vi "Dresden R2R Sputter 03.02.2018 IY24.vi"() -> ()   [LabVIEW 2009] (continued)
                                stop <- w22715 stop-if-true
                                n21716 = Greater?(x=w22721, y=50) -> (0:w22719:bool)
                                n21717 = case shown="True" w22719 {
                                frame #0 {
                                }
                                frame #1 {
                                n21718 = local write "Semi"(TRUE ("Semi")) -> ()
                                n21719 = local write "Error Message"("Start up process  cancelled\nbecause MP not stopped.\nPlease check MP4 connections." ("Error Message")) -> ()
                                }
                                }
                                n21720 = local read "Ch4_Mp_di"() -> (w22718:bool)
                                n21721 = case shown="True" w22718 {
                                tunnel: [TRUE FALSE] -> w22717
                                frame #0 {
                                }
                                frame #1 {
                                n21722 = Wait Until Next ms Multiple(millisecond multiple=u32 200) -> ()  [unwired: 1 out]
                                n21723 = local write "Ch4_Mp_do"(FALSE ("Ch1_Tp_bv_do")) -> ()
                                }
                                }
                                n21724 = local read "Semi"() -> (w22716:bool)
                                n21725 = Or(x=w22717, y=w22716) -> (x .or. y?=w22715:bool)
                                }
                                }
                                frame #1 {
                                }
                                }
                                }
                                frame #1 {
                                n21726 = local read "Semi"() -> (w22728:bool)
                                n21727 = case shown="False" w22728 {
                                frame #0 {
                                n21728 = local write "Ch4_PA10"(TRUE ("PA3")) -> ()
                                n21729 = Wait Until Next ms Multiple(millisecond multiple=u32 1000) -> ()  [unwired: 1 out]
                                }
                                frame #1 {
                                }
                                }
                                }
                                }
                              }
                              frame #1 {
                              }
                            }
                          }
                          frame #6 {
                            # "OPEN PL-VBV1"
                            n21730 = local read "Semi"() -> (w22731:bool)
                            n21731 = case shown="False" w22731 {
                              frame #0 {
                                n21732 = stacked-sequence {
                                frame #0 {
                                n21733 = local read "Semi"() -> (w22732:bool)
                                n21734 = case shown="False" w22732 {
                                frame #0 {
                                n21735 = while {
                                i -> [w22739]
                                stop <- w22734 stop-if-true
                                n21736 = Greater?(x=w22739, y=50) -> (0:w22737:bool)
                                n21737 = case shown="True" w22737 {
                                frame #0 {
                                }
                                frame #1 {
                                n21738 = local write "Semi"(TRUE ("Semi")) -> ()
                                n21739 = local write "Error Message"("Start up process  cancelled\nbecause  PL-VBV not opened.\nPlease check PL-VBV4 connections." ("Error Message")) -> ()
                                }
                                }
                                n21740 = local read "Ch4_Pl_atm_di"() -> (w22733:bool)
                                n21741 = case shown="False" w22733 {
                                tunnel: [w22741 TRUE] -> w22736
                                frame #0 {
                                n21742 = local read "Ch4_Pl_vbv_di"() -> (w22740:bool)
                                n21743 = case shown="False" w22740 {
                                tunnel: [FALSE TRUE] -> w22741
                                frame #0 {
                                n21744 = local write "Ch4_Pl_vbv_do"(TRUE ("Ch1_Tp_bv_do")) -> ()
                                n21745 = Wait Until Next ms Multiple(millisecond multiple=u32 200) -> ()  [unwired: 1 out]
                                }
                                frame #1 {
                                }
                                }
                                }
                                frame #1 {
                                }
                                }
                                n21746 = local read "Semi"() -> (w22735:bool)
                                n21747 = Or(x=w22736, y=w22735) -> (x .or. y?=w22734:bool)
                                }
                                }
                                frame #1 {
                                }
                                }
                                }
                                frame #1 {
                                n21748 = local read "Semi"() -> (w22749:bool)
                                n21749 = case shown="False" w22749 {
                                frame #0 {
                                n21750 = local write "Ch4_PA11"(TRUE ("PA3")) -> ()
                                n21751 = Wait Until Next ms Multiple(millisecond multiple=u32 1000) -> ()  [unwired: 1 out]
                                }
                                frame #1 {
                                }
                                }
                                }
                                }
                              }
                              frame #1 {
                              }
                            }
                          }
                          frame #7 {
                            # "CHECK PL-PRESSURE"
                            n21752 = local read "Semi"() -> (w22752:bool)
                            n21753 = case shown="False" w22752 {
                              frame #0 {
                                n21754 = stacked-sequence {
                                frame #0 {
                                n21755 = local read "Semi"() -> (w22753:bool)
                                n21756 = case shown="False" w22753 {
                                frame #0 {
                                n21757 = while {
                                i -> [w22760]
                                stop <- w22755 stop-if-true
                                n21758 = Greater?(x=w22760, y=50) -> (0:w22758:bool)
                                n21759 = case shown="True" w22758 {
                                frame #0 {
                                }
                                frame #1 {
                                n21760 = local write "Semi"(TRUE ("Semi")) -> ()
                                n21761 = local write "Error Message"("Start up process  cancelled\nbecause  PL-ATM not opened.\nPlease check PL-ATM connections." ("Error Message")) -> ()
                                }
                                }
                                n21762 = local read "Ch4_Pl_atm_di"() -> (w22754:bool)
                                n21763 = case shown="True" w22754 {
                                tunnel: [FALSE TRUE] -> w22757
                                frame #0 {
                                }
                                frame #1 {
                                n21764 = Wait Until Next ms Multiple(millisecond multiple=u32 500) -> ()  [unwired: 1 out]
                                }
                                }
                                n21765 = local read "Semi"() -> (w22756:bool)
                                n21766 = Or(x=w22757, y=w22756) -> (x .or. y?=w22755:bool)
                                }
                                }
                                frame #1 {
                                }
                                }
                                }
                                frame #1 {
                                n21767 = local read "Semi"() -> (w22766:bool)
                                n21768 = case shown="False" w22766 {
                                frame #0 {
                                n21769 = local write "Ch4_PA12"(TRUE ("PA3")) -> ()
                                n21770 = Wait Until Next ms Multiple(millisecond multiple=u32 1000) -> ()  [unwired: 1 out]
                                }
                                frame #1 {
                                }
                                }
                                }
                                }
                              }
                              frame #1 {
                              }
                            }
                          }
                          frame #8 {
                            # "False CH-ATM"
                            n21771 = local read "Semi"() -> (w22769:bool)
                            n21772 = case shown="False" w22769 {
                              frame #0 {
                                n21773 = stacked-sequence {
                                frame #0 {
                                n21774 = local read "Semi"() -> (w22770:bool)
                                n21775 = case shown="False" w22770 {
                                frame #0 {
                                n21776 = local write "Ch4_Ch_atm_do"(FALSE ("Ch1_Pl_atm_do")) -> ()
                                }
                                frame #1 {
                                }
                                }
                                }
                                frame #1 {
                                n21777 = local read "Semi"() -> (w22772:bool)
                                n21778 = case shown="False" w22772 {
                                frame #0 {
                                n21779 = local write "Ch4_PA13"(TRUE ("PA3")) -> ()
                                n21780 = Wait Until Next ms Multiple(millisecond multiple=u32 1000) -> ()  [unwired: 1 out]
                                }
                                frame #1 {
                                }
                                }
                                }
                                }
                              }
                              frame #1 {
                              }
                            }
                          }
                          frame #9 {
                            # "OPEN PC-BV"
                            n21781 = local read "Semi"() -> (w22775:bool)
                            n21782 = case shown="False" w22775 {
                              frame #0 {
                                n21783 = stacked-sequence {
                                frame #0 {
                                n21784 = local read "Semi"() -> (w22776:bool)
                                n21785 = case shown="False" w22776 {
                                frame #0 {
                                n21786 = stacked-sequence {
                                frame #0 {
                                n21787 = local read "Semi"() -> (w22777:bool)
                                n21788 = case shown="False" w22777 {
                                frame #0 {
                                n21789 = local write "Pc_bv4_auto_open"(TRUE ("Tp1_auto_start")) -> ()
                                }
                                frame #1 {
                                }
                                }
                                }
                                frame #1 {
                                n21790 = local read "Semi"() -> (w22779:bool)
                                n21791 = case shown="False" w22779 {
                                frame #0 {
                                n21792 = Wait (ms)(milliseconds to wait=u32 1000) -> ()  [unwired: 1 out]
                                }
                                frame #1 {
                                }
                                }
                                }
                                frame #2 {
                                n21793 = local read "Semi"() -> (w22781:bool)
                                n21794 = case shown="False" w22781 {
                                frame #0 {
                                n21795 = while {
                                i -> [w22787]
                                stop <- w22783 stop-if-true
                                n21796 = local read "Pc_bv_opened_ch4"() -> (w22785:bool)
                                n21797 = Greater?(x=w22787, y=120) -> (0:w22786:bool)
                                n21798 = local read "Semi"() -> (w22784:bool)
                                n21799 = Compound Arithmetic op=OR(w22784, w22785, w22786) -> (w22783:bool)
                                n21800 = Wait (ms)(milliseconds to wait=u32 500) -> ()  [unwired: 1 out]
                                }
                                }
                                frame #1 {
                                }
                                }
                                }
                                frame #3 {
                                n21801 = local read "Semi"() -> (w22789:bool)
                                n21802 = case shown="False" w22789 {
                                frame #0 {
                                n21803 = local read "Pc_bv_opened_ch4"() -> (w22790:bool)
                                n21804 = case shown="False" w22790 {
                                frame #0 {
                                n21805 = local write "Pc_bv4_auto_open"(TRUE ("Pc_bv1_auto_open")) -> ()
                                }
                                frame #1 {
                                }
                                }
                                }
                                frame #1 {
                                }
                                }
                                }
                                frame #4 {
                                n21806 = local read "Semi"() -> (w22792:bool)
                                n21807 = case shown="False" w22792 {
                                frame #0 {
                                n21808 = local read "Pc_bv_opened_ch4"() -> (w22793:bool)
                                n21809 = case shown="False" w22793 {
                                frame #0 {
                                n21810 = Wait (ms)(milliseconds to wait=u32 1000) -> ()  [unwired: 1 out]
                                }
                                frame #1 {
                                }
                                }
                                }
                                frame #1 {
                                }
                                }
                                }
                                frame #5 {
                                n21811 = local read "Semi"() -> (w22795:bool)
                                n21812 = case shown="False" w22795 {
                                frame #0 {
                                n21813 = while {
                                i -> [w22801]
                                stop <- w22797 stop-if-true
                                n21814 = local read "Pc_bv_opened_ch4"() -> (w22799:bool)
                                n21815 = Greater?(x=w22801, y=120) -> (0:w22800:bool)
                                n21816 = local read "Semi"() -> (w22798:bool)
                                n21817 = Compound Arithmetic op=OR(w22798, w22799, w22800) -> (w22797:bool)
                                n21818 = Wait (ms)(milliseconds to wait=u32 500) -> ()  [unwired: 1 out]
                                }
                                }
                                frame #1 {
                                }
                                }
                                }
                                frame #6 {
                                n21819 = local read "Semi"() -> (w22803:bool)
                                n21820 = case shown="False" w22803 {
                                frame #0 {
                                n21821 = local read "Pc_bv_opened_ch4"() -> (w22804:bool)
                                n21822 = case shown="False" w22804 {
                                frame #0 {
                                n21823 = local write "Error Message"("Start up process  cancelled\nbecause  PC-BV not opened.\nPlease check PC-BV4 connections." ("Error Message")) -> ()
                                n21824 = Wait (ms)(milliseconds to wait=u32 1000) -> ()  [unwired: 1 out]
                                }
                                frame #1 {
                                }
                                }
                                }
                                frame #1 {
                                }
                                }
                                }
                                }
                                }
                                frame #1 {
                                }
                                }
                                }
                                frame #1 {
                                n21825 = local read "Semi"() -> (w22807:bool)
                                n21826 = case shown="False" w22807 {
                                frame #0 {
                                n21827 = Wait Until Next ms Multiple(millisecond multiple=u32 1000) -> ()  [unwired: 1 out]
                                n21828 = local write "Ch4_PA14"(TRUE ("PA3")) -> ()
                                }
                                frame #1 {
                                }
                                }
                                }
                                }
                              }
                              frame #1 {
                              }
                            }
                          }
                          frame #10 {
                            # "OPEN CH-VBV"
                            n21829 = local read "Semi"() -> (w22810:bool)
                            n21830 = case shown="False" w22810 {
                              frame #0 {
                                n21831 = stacked-sequence {
                                frame #0 {
                                n21832 = local read "Semi"() -> (w22811:bool)
                                n21833 = case shown="False" w22811 {
                                frame #0 {
                                n21834 = while {
                                i -> [w22818]
                                stop <- w22813 stop-if-true
                                n21835 = Greater?(x=w22818, y=200) -> (0:w22816:bool)
                                n21836 = case shown="True" w22816 {
                                frame #0 {
                                }
                                frame #1 {
                                n21837 = local write "Semi"(TRUE ("Semi")) -> ()
                                n21838 = local write "Error Message"("Start up process  cancelled\nbecause  CH-VBV not opened.\nPlease check  CH-VBV connections." ("Error Message")) -> ()
                                }
                                }
                                n21839 = local read "Ch4_Ch_atm_di"() -> (w22812:bool)
                                n21840 = case shown="False" w22812 {
                                tunnel: [w22819 TRUE] -> w22815
                                frame #0 {
                                n21841 = local read "Ch4_Ch_vbv_di"() -> (w22820:bool)
                                n21842 = case shown="False" w22820 {
                                tunnel: [FALSE TRUE] -> w22819
                                frame #0 {
                                n21843 = local write "Ch4_Ch_vbv_do"(TRUE ("Ch1_Tp_bv_do")) -> ()
                                n21844 = Wait Until Next ms Multiple(millisecond multiple=u32 200) -> ()  [unwired: 1 out]
                                }
                                frame #1 {
                                }
                                }
                                }
                                frame #1 {
                                }
                                }
                                n21845 = local read "Semi"() -> (w22814:bool)
                                n21846 = Or(x=w22815, y=w22814) -> (x .or. y?=w22813:bool)
                                }
                                }
                                frame #1 {
                                }
                                }
                                }
                                frame #1 {
                                n21847 = local read "Semi"() -> (w22828:bool)
                                n21848 = case shown="False" w22828 {
                                frame #0 {
                                n21849 = local write "Ch4_PA15"(TRUE ("PA3")) -> ()
                                n21850 = Wait Until Next ms Multiple(millisecond multiple=u32 1000) -> ()  [unwired: 1 out]
                                }
                                frame #1 {
                                }
                                }
                                }
                                }
                              }
                              frame #1 {
                              }
                            }
                          }
                          frame #11 {
                            # "OPEN/CLOSE TRNS GV-BP"
                            n21851 = local read "Semi"() -> (w22831:bool)
                            n21852 = case shown="False" w22831 {
                              frame #0 {
                                n21853 = stacked-sequence {
                                frame #0 {
                                n21854 = local read "Semi"() -> (w22832:bool)
                                n21855 = case shown="False" w22832 {
                                frame #0 {
                                n21856 = while {
                                i -> [w22841]
                                stop <- w22836 stop-if-true
                                n21857 = Greater?(x=w22841, y=800) -> (0:w22839:bool)
                                n21858 = case shown="True" w22839 {
                                frame #0 {
                                }
                                frame #1 {
                                n21859 = local read "Ch3_pressure"() -> (w22861:dbl)
                                n21860 = Less?(x=w22861, y=1) -> (x < y?=w22860:bool)
                                n21861 = case shown="True" w22860 {
                                frame #0 {
                                n21862 = local write "Error Message"("Start up process  cancelled\nbecause \n Trns GV-BP not closed.\nPlease check \nTrns GV-BP connections." ("Error Message")) -> ()
                                }
                                frame #1 {
                                n21863 = local write "Error Message"("Start up process  cancelled\nbecause \n Trns GV-BP not opened.\nPlease check \nTrns GV-BP connections." ("Error Message")) -> ()
                                }
                                }
                                n21864 = local write "Semi"(TRUE ("Semi")) -> ()
                                }
                                }
                                n21865 = local read "Ch3_pressure"() -> (w22835:dbl)
                                n21866 = Less?(x=w22835, y=1) -> (x < y?=w22833:bool)
                                n21867 = case shown="True" w22833 {
                                tunnel: [w22843 w22851] -> w22838
                                frame #0 {
                                n21868 = local read "Ch4_Trns_gv_bp_di"() -> (w22842:bool)
                                n21869 = case shown="True" w22842 {
                                tunnel: [TRUE FALSE] -> w22843
                                frame #0 {
                                }
                                frame #1 {
                                n21870 = local write "Ch4_Trns_gv_bp_do"(FALSE ("Ch1_Tp_bv_do")) -> ()
                                n21871 = Wait Until Next ms Multiple(millisecond multiple=u32 200) -> ()  [unwired: 1 out]
                                }
                                }
                                }
                                frame #1 {
                                n21872 = local read "Ch4pressure"() -> (w22850:dbl)
                                n21873 = Greater Or Equal?(x=w22850, y=700.0) -> (x >= y?=w22848:bool)
                                n21874 = case shown="True" w22848 {
                                tunnel: [FALSE w22855] -> w22851
                                frame #0 {
                                n21875 = Wait Until Next ms Multiple(millisecond multiple=u32 500) -> ()  [unwired: 1 out]
                                }
                                frame #1 {
                                n21876 = local read "Ch4_Trns_gv_bp_di"() -> (w22854:bool)
                                n21877 = case shown="False" w22854 {
                                tunnel: [FALSE TRUE] -> w22855
                                frame #0 {
                                n21878 = local write "Ch4_Trns_gv_bp_do"(TRUE ("Ch1_Tp_bv_do")) -> ()
                                n21879 = Wait Until Next ms Multiple(millisecond multiple=u32 200) -> ()  [unwired: 1 out]
                                }
                                frame #1 {
                                }
                                }
                                }
                                }
                                }
                                }
                                n21880 = local read "Semi"() -> (w22837:bool)
                                n21881 = Or(x=w22838, y=w22837) -> (x .or. y?=w22836:bool)
                                }
                                }
                                frame #1 {
                                }
                                }
                                }
                                frame #1 {
                                n21882 = local read "Semi"() -> (w22866:bool)
                                n21883 = case shown="False" w22866 {
                                frame #0 {
                                n21884 = local write "Ch4_PA16"(TRUE ("PA3")) -> ()
                                n21885 = Wait Until Next ms Multiple(millisecond multiple=u32 1000) -> ()  [unwired: 1 out]
                                }
                                frame #1 {
                                }
                                }
                                }
                                }
                              }
                              frame #1 {
                              }
                            }
                          }
                          frame #12 {
                            # "CHECK CH-ATM"
                            n21886 = local read "Semi"() -> (w22869:bool)
                            n21887 = case shown="False" w22869 {
                              frame #0 {
                                n21888 = stacked-sequence {
                                frame #0 {
                                n21889 = local read "Semi"() -> (w22870:bool)
                                n21890 = case shown="False" w22870 {
                                frame #0 {
                                n21891 = while {
                                i -> [w22877]
                                stop <- w22872 stop-if-true
                                n21892 = Greater?(x=w22877, y=1200) -> (0:w22875:bool)
                                n21893 = case shown="True" w22875 {
                                frame #0 {
                                }
                                frame #1 {
                                n21894 = local write "Semi"(TRUE ("Semi")) -> ()
                                n21895 = local write "Error Message"("Start up process  cancelled\nbecause  CH-ATM not opened.\nPlease check CH-ATM connections." ("Error Message")) -> ()
                                }
                                }
                                n21896 = local read "Ch4_Ch_atm_di"() -> (w22871:bool)
                                n21897 = case shown="False" w22871 {
                                tunnel: [FALSE TRUE] -> w22874
                                frame #0 {
                                n21898 = Wait Until Next ms Multiple(millisecond multiple=u32 500) -> ()  [unwired: 1 out]
                                }
                                frame #1 {
                                }
                                }
                                n21899 = local read "Semi"() -> (w22873:bool)
                                n21900 = Or(x=w22874, y=w22873) -> (x .or. y?=w22872:bool)
                                }
                                }
                                frame #1 {
                                }
                                }
                                }
                                frame #1 {
                                n21901 = local read "Semi"() -> (w22883:bool)
                                n21902 = case shown="False" w22883 {
                                frame #0 {
                                n21903 = local write "Ch4_PA17"(TRUE ("PA3")) -> ()
                                n21904 = Wait Until Next ms Multiple(millisecond multiple=u32 1000) -> ()  [unwired: 1 out]
                                }
                                frame #1 {
                                }
                                }
                                }
                                }
                              }
                              frame #1 {
                              }
                            }
                          }
                          frame #13 {
                            # "CLOSE CH-VBV"
                            n21905 = local read "Semi"() -> (w22886:bool)
                            n21906 = case shown="False" w22886 {
                              frame #0 {
                                n21907 = stacked-sequence {
                                frame #0 {
                                n21908 = local read "Semi"() -> (w22887:bool)
                                n21909 = case shown="False" w22887 {
                                frame #0 {
                                n21910 = while {
                                i -> [w22894]
                                stop <- w22888 stop-if-true
                                n21911 = Greater?(x=w22894, y=50) -> (0:w22892:bool)
                                n21912 = case shown="True" w22892 {
                                frame #0 {
                                }
                                frame #1 {
                                n21913 = local write "Semi"(TRUE ("Semi")) -> ()
                                n21914 = local write "Error Message"("Start up process  cancelled\nbecause  CH-VBV not closed.\nPlease check  CH-VBV connections." ("Error Message")) -> ()
                                }
                                }
                                n21915 = local read "Ch4_Ch_vbv_di"() -> (w22891:bool)
                                n21916 = case shown="True" w22891 {
                                tunnel: [TRUE FALSE] -> w22890
                                frame #0 {
                                }
                                frame #1 {
                                n21917 = Wait Until Next ms Multiple(millisecond multiple=u32 200) -> ()  [unwired: 1 out]
                                n21918 = local write "Ch4_Ch_vbv_do"(FALSE ("Ch1_Tp_bv_do")) -> ()
                                }
                                }
                                n21919 = local read "Semi"() -> (w22889:bool)
                                n21920 = Or(x=w22890, y=w22889) -> (x .or. y?=w22888:bool)
                                }
                                }
                                frame #1 {
                                }
                                }
                                }
                                frame #1 {
                                n21921 = local read "Semi"() -> (w22901:bool)
                                n21922 = case shown="False" w22901 {
                                frame #0 {
                                n21923 = local write "Ch4_PA18"(TRUE ("PA3")) -> ()
                                n21924 = Wait Until Next ms Multiple(millisecond multiple=u32 1000) -> ()  [unwired: 1 out]
                                }
                                frame #1 {
                                }
                                }
                                }
                                }
                              }
                              frame #1 {
                              }
                            }
                          }
                          frame #14 {
                            # "Close PL-VBV"
                            n21925 = local read "Semi"() -> (w22904:bool)
                            n21926 = case shown="False" w22904 {
                              frame #0 {
                                n21927 = stacked-sequence {
                                frame #0 {
                                n21928 = local read "Semi"() -> (w22905:bool)
                                n21929 = case shown="False" w22905 {
                                frame #0 {
                                n21930 = while {
                                i -> [w22912]
                                stop <- w22906 stop-if-true
                                n21931 = Greater?(x=w22912, y=50) -> (0:w22910:bool)
                                n21932 = case shown="True" w22910 {
                                frame #0 {
                                }
                                frame #1 {
                                n21933 = local write "Semi"(TRUE ("Semi")) -> ()
                                n21934 = local write "Error Message"("Start up process  cancelled\nbecause  PL-VBV not closed.\nPlease check PL-VBV connections." ("Error Message")) -> ()
                                }
                                }
                                n21935 = local read "Ch4_Pl_vbv_di"() -> (w22909:bool)
                                n21936 = case shown="True" w22909 {
                                tunnel: [TRUE FALSE] -> w22908
                                frame #0 {
                                }
                                frame #1 {
                                n21937 = Wait Until Next ms Multiple(millisecond multiple=u32 200) -> ()  [unwired: 1 out]
                                n21938 = local write "Ch4_Pl_vbv_do"(FALSE ("Ch1_Tp_bv_do")) -> ()
                                }
                                }
                                n21939 = local read "Semi"() -> (w22907:bool)
                                n21940 = Or(x=w22908, y=w22907) -> (x .or. y?=w22906:bool)
                                }
                                }
                                frame #1 {
                                }
                                }
                                }
                                frame #1 {
                                n21941 = local read "Semi"() -> (w22919:bool)
                                n21942 = case shown="False" w22919 {
                                frame #0 {
                                n21943 = local write "Ch4_PA19"(TRUE ("PA3")) -> ()
                                n21944 = Wait Until Next ms Multiple(millisecond multiple=u32 1000) -> ()  [unwired: 1 out]
                                }
                                frame #1 {
                                }
                                }
                                }
                                }
                              }
                              frame #1 {
                              }
                            }
                          }
                          frame #15 {
                            # "OPEN TP-BV"
                            n21945 = local read "Semi"() -> (w22922:bool)
                            n21946 = case shown="False" w22922 {
                              frame #0 {
                                n21947 = stacked-sequence {
                                frame #0 {
                                n21948 = local read "Semi"() -> (w22923:bool)
                                n21949 = case shown="False" w22923 {
                                frame #0 {
                                n21950 = while {
                                i -> [w22930]
                                stop <- w22925 stop-if-true
                                n21951 = Greater?(x=w22930, y=50) -> (0:w22928:bool)
                                n21952 = case shown="True" w22928 {
                                frame #0 {
                                }
                                frame #1 {
                                n21953 = local write "Semi"(TRUE ("Semi")) -> ()
                                n21954 = local write "Error Message"("Start up process  cancelled\nbecause  TP-BV not opened.\nPlease check TP-BV4 connections." ("Error Message")) -> ()
                                }
                                }
                                n21955 = local read "Ch4_Tp_bv_di"() -> (w22924:bool)
                                n21956 = case shown="False" w22924 {
                                tunnel: [FALSE TRUE] -> w22927
                                frame #0 {
                                n21957 = Wait Until Next ms Multiple(millisecond multiple=u32 200) -> ()  [unwired: 1 out]
                                n21958 = local write "Ch4_Tp_bv_do"(TRUE ("Ch1_Tp_bv_do")) -> ()
                                }
                                frame #1 {
                                }
                                }
                                n21959 = local read "Semi"() -> (w22926:bool)
                                n21960 = Or(x=w22927, y=w22926) -> (x .or. y?=w22925:bool)
                                }
                                }
                                frame #1 {
                                }
                                }
                                }
                                frame #1 {
                                n21961 = local read "Semi"() -> (w22937:bool)
                                n21962 = case shown="False" w22937 {
                                frame #0 {
                                n21963 = local write "Ch4_PA20"(TRUE ("PA3")) -> ()
                                n21964 = Wait Until Next ms Multiple(millisecond multiple=u32 1000) -> ()  [unwired: 1 out]
                                }
                                frame #1 {
                                }
                                }
                                }
                                }
                              }
                              frame #1 {
                              }
                            }
                          }
                          frame #16 {
                            # "CLOSE CH-ATM"
                            n21965 = local read "Semi"() -> (w22940:bool)
                            n21966 = case shown="False" w22940 {
                              frame #0 {
                                n21967 = stacked-sequence {
                                frame #0 {
                                n21968 = local read "Semi"() -> (w22941:bool)
                                n21969 = case shown="False" w22941 {
                                frame #0 {
                                n21970 = while {
                                i -> [w22948]
                                stop <- w22942 stop-if-true
                                n21971 = Greater?(x=w22948, y=50) -> (0:w22946:bool)
                                n21972 = case shown="True" w22946 {
                                frame #0 {
                                }
                                frame #1 {
                                n21973 = local write "Semi"(TRUE ("Semi")) -> ()
                                n21974 = local write "Error Message"("Start up process  cancelled\nbecause CH-ATM not closed.\nPlease check CH-ATM connections." ("Error Message")) -> ()
                                }
                                }
                                n21975 = local read "Ch4_Ch_atm_di"() -> (w22945:bool)
                                n21976 = case shown="True" w22945 {
                                tunnel: [TRUE FALSE] -> w22944
                                frame #0 {
                                }
                                frame #1 {
                                n21977 = Wait Until Next ms Multiple(millisecond multiple=u32 200) -> ()  [unwired: 1 out]
                                n21978 = local write "Ch4_Ch_atm_do"(TRUE ("Ch1_Tp_bv_do")) -> ()
                                }
                                }
                                n21979 = local read "Semi"() -> (w22943:bool)
                                n21980 = Or(x=w22944, y=w22943) -> (x .or. y?=w22942:bool)
                                }
                                }
                                frame #1 {
                                }
                                }
                                }
                                frame #1 {
                                n21981 = local read "Semi"() -> (w22955:bool)
                                n21982 = case shown="False" w22955 {
                                frame #0 {
                                n21983 = local write "Ch4_PA21"(TRUE ("PA3")) -> ()
                                n21984 = Wait Until Next ms Multiple(millisecond multiple=u32 1000) -> ()  [unwired: 1 out]
                                }
                                frame #1 {
                                }
                                }
                                }
                                }
                              }
                              frame #1 {
                              }
                            }
                          }
                          frame #17 {
                            # "CLOSE PL-ATM"
                            n21985 = local read "Semi"() -> (w22958:bool)
                            n21986 = case shown="False" w22958 {
                              frame #0 {
                                n21987 = stacked-sequence {
                                frame #0 {
                                n21988 = local read "Semi"() -> (w22959:bool)
                                n21989 = case shown="False" w22959 {
                                frame #0 {
                                n21990 = while {
                                i -> [w22966]
                                stop <- w22960 stop-if-true
                                n21991 = Greater?(x=w22966, y=50) -> (0:w22964:bool)
                                n21992 = case shown="True" w22964 {
                                frame #0 {
                                }
                                frame #1 {
                                n21993 = local write "Semi"(TRUE ("Semi")) -> ()
                                n21994 = local write "Error Message"("Start up process  cancelled\nbecause  PL-ATM not closed.\nPlease check PL-ATM4 connections." ("Error Message")) -> ()
                                }
                                }
                                n21995 = local read "Ch4_Pl_atm_di"() -> (w22963:bool)
                                n21996 = case shown="True" w22963 {
                                tunnel: [TRUE FALSE] -> w22962
                                frame #0 {
                                }
                                frame #1 {
                                n21997 = Wait Until Next ms Multiple(millisecond multiple=u32 200) -> ()  [unwired: 1 out]
                                n21998 = local write "Ch4_Pl_atm_do"(TRUE ("Ch1_Tp_bv_do")) -> ()
                                }
                                }
                                n21999 = local read "Semi"() -> (w22961:bool)